vi "HFRR ADV v038 new software.vi"() -> ()   [LabVIEW 2025] (continued)
            n2186 = String Subset(string=w2638, length (rest)=9 ("length (rest)")) -> (substring=w2640:string)  [unwired: 1 in]
            n2187 = String Subset(string=w2615, length (rest)=6 ("length (rest)")) -> (substring=w2617:string)  [unwired: 1 in]
            n2188 = String Subset(string=w2633, length (rest)=9 ("length (rest)")) -> (substring=w2635:string)  [unwired: 1 in]
            n2189 = String Subset(string=w2611, length (rest)=6 ("length (rest)")) -> (substring=w2613:string)  [unwired: 1 in]
            n2190 = String Subset(string=w2628, length (rest)=9 ("length (rest)")) -> (substring=w2630:string)  [unwired: 1 in]
            n2191 = String Subset(string=w2607, length (rest)=6 ("length (rest)")) -> (substring=w2609:string)  [unwired: 1 in]
            n2192 = String Subset(string=w2623, length (rest)=9 ("length (rest)")) -> (substring=w2625:string)  [unwired: 1 in]
            n2193 = Fract/Exp String To Number(string=w2621) -> (number=w2601:dbl)  [unwired: 3 in, 1 out]
            n2194 = Fract/Exp String To Number(string=w2640) -> (number=w2641:dbl)  [unwired: 3 in, 1 out]
            n2195 = Fract/Exp String To Number(string=w2617) -> (number=w2600:dbl)  [unwired: 3 in, 1 out]
            n2196 = Fract/Exp String To Number(string=w2635) -> (number=w2636:dbl)  [unwired: 3 in, 1 out]
            n2197 = Fract/Exp String To Number(string=w2613) -> (number=w2599:dbl)  [unwired: 3 in, 1 out]
            n2198 = Fract/Exp String To Number(string=w2630) -> (number=w2631:dbl)  [unwired: 3 in, 1 out]
            n2199 = Fract/Exp String To Number(string=w2609) -> (number=w2598:dbl)  [unwired: 3 in, 1 out]
            n2200 = Fract/Exp String To Number(string=w2625) -> (number=w2626:dbl)  [unwired: 3 in, 1 out]
            n2201 = local write "sample1"(w2601) -> ()
            n2202 = local write "freq1"(w2641) -> ()
            n2203 = local write "sample2"(w2600) -> ()
            n2204 = local write "freq2"(w2636) -> ()
            n2205 = local write "sample3"(w2599) -> ()
            n2206 = local write "freq3"(w2631) -> ()
            n2207 = local write "sample4"(w2598) -> ()
            n2208 = local write "freq 4"(w2626) -> ()
          }
        }
      }
    }
    n2209 = case shown="True" w2199 {
      selector: w2199 -> [_ w2218]
      frame False {
      }
      frame True {
        n2210 = Not(x=w2218) -> (.not. x?=w2214:bool)
        n2211 = local write "service 3"(w2214) -> ()
        n2212 = local write "OPEN 6"(w2214) -> ()
        n2213 = call <vilib>:"System Exec.vi"("wait until completion? (T)"=TRUE, "command line"="C:\\LAB-IQ\\Scar View.exe") -> ("error out"=→"error out 5":errorcluster)  [unwired: 6 in, 3 out]
      }
    }
    n2214 = case shown="\"Acquire\", Default" w2208 {
      frame "Acquire", Default {
        # "Elapsed time\ncof\nstroke\nAir temp\nTemp\nHumidity"
        n2215 = disable-structure shown="Disabled" {
          frame Disabled {
            n2216 = local read "Flag"() -> (w2917:dbl)
            n2217 = local read "RUN"() -> (w2914:bool)
            n2218 = Not(x=w2914) -> (.not. x?=w2913:bool)
            n2219 = Equal?(x=w2917, y=10.0) -> (x = y?=w2915:bool)
            n2220 = And(x=w2915, y=w2913) -> (x .and. y?=w2912:bool)
            n2221 = case shown="True" w2912 {
              frame False {
              }
              frame True {
                w2918 = FALSE ("Heater Button")
                n2222 = local write "Humidity"(w2918) -> ()
                n2223 = local write "Heater Button"(w2918) -> ()
              }
            }
          }
          frame Enabled {
          }
        }
        n2224 = disable-structure shown="Disabled" {
          frame Disabled {
            n2225 = case shown="True" {
              selector: _ -> [_ _]
              frame False {
              }
              frame True {
                w2967 = TRUE ("Heater")
                n2226 = local write "Humidity"(w2967) -> ()
                n2227 = local write "Heater Button"(w2967) -> ()
                n2228 = local read "TEST STANDARD"() -> (w2970:T3)
                n2229 = local read "TEST STANDARD"() -> (w2965:T3)
                n2230 = Equal?(x=w2970, y=enum16{"ASTM D6079", "ISO 12156", "Custom"}."ISO 12156" ("Test Standard")) -> (x = y?=w2968:bool)
                n2231 = Equal?(x=w2965, y=enum16{"ASTM D6079", "ISO 12156", "Custom"}."ASTM D6079" ("Test Standard")) -> (x = y?=w2964:bool)
                n2232 = case shown="True" w2968 {
                  frame False {
                  }
                  frame True {
                    n2233 = local write "airtempflg"(FALSE ("airtempflg")) -> ()
                    n2234 = local write item#-1(TRUE ("Heater")) -> ()
                  }
                }
                n2235 = case shown="True" w2964 {
                  frame False {
                  }
                  frame True {
                    n2236 = local write "airtempflg"(TRUE ("airtempflg")) -> ()
                    n2237 = local write item#-1(FALSE ("Heater")) -> ()
                  }
                }
              }
            }
          }
          frame Enabled {
          }
        }
        n2238 = stacked-sequence {
          frame #0 {
            n2239 = case shown="True" "RST FF" {
              frame False {
              }
              frame True {
                w2984 = 0.0 ("X Scale.Range:Maximum")
                n2240 = property on="Frictional Force ( N )" class="WFChart (strict)"("XScale.Maximum"=600.0 ("X Scale.Range:Maximum"), "XScale.Minimum"=w2984, "YScale.Maximum"=10.0 ("Y Scale.Range:Maximum"), "YScale.Minimum"=w2984) -> ()  [unwired: 2 in, 2 out]
              }
            }
          }
          frame #1 {
            n2241 = case shown="True" "RST TEMP" {
              frame False {
              }
              frame True {
                n2242 = property on="Temperature ( Deg C )" class="WFChart (strict)"("XScale.Minimum"=0.0 ("X Scale.Range:Minimum"), "XScale.Maximum"=600.0 ("X Scale.Range:Maximum"), "YScale.Minimum"=0.0 ("Y Scale.Range:Minimum"), "YScale.Maximum"=100.0 ("Y Scale.Range:Maximum")) -> ()  [unwired: 2 in, 2 out]
              }
            }
          }
          frame #2 {
            n2243 = case shown="True" "RSTCOF" {
              frame False {
              }
              frame True {
                n2244 = property on="Coefficient of Friction" class="WFChart (strict)"("XScale.Minimum"=0.0 ("X Scale.Range:Minimum"), "XScale.Maximum"=600.0 ("X Scale.Range:Maximum"), "YScale.Maximum"=1.0 ("X Scale.Range:Minimum"), "YScale.Minimum"=0.0 ("X Scale.Range:Minimum")) -> ()  [unwired: 2 in, 2 out]
              }
            }
          }
          frame #3 {
            n2245 = case shown="True" "RSTCOF 2" {
              frame False {
              }
              frame True {
                (unwired) 100.0 ("Y Scale.Range:Maximum")
                (unwired) 0.0 ("Y Scale.Range:Minimum")
                (unwired) 600.0 ("X Scale.Range:Maximum")
                (unwired) 0.0 ("X Scale.Range:Minimum")
              }
            }
          }
          frame #4 {
            n2246 = case shown="True" "RSTCOF 3" {
              frame False {
              }
              frame True {
                n2247 = property on="Electrical Contact Resistance ( % )" class="WFChart (strict)"("XScale.Minimum"=0.0 ("X Scale.Range:Minimum"), "XScale.Maximum"=600.0 ("X Scale.Range:Maximum"), "YScale.Minimum"=0.0 ("Y Scale.Range:Minimum"), "YScale.Maximum"=100.0 ("Y Scale.Range:Maximum")) -> ()  [unwired: 2 in, 2 out]
              }
            }
          }
        }
        n2248 = local read "RUN"() -> (w2907:bool)
        n2249 = case shown="False" w2907 {
          frame False {
          }
          frame True {
          }
        }
        n2250 = local read "RUN"() -> (w2911:bool)
        n2251 = case shown="False" w2911 {
          tunnel: [FALSE ("TEST RUNNING") TRUE ("TEST RUNNING")] -> w2910
          frame False {
            w3003 = 0.0 ("Flag")
            n2252 = local write "Elapsed time"(0.0 ("elapsedtime")) -> ()
            n2253 = local write "Time Remaining"(w3003) -> ()
            n2254 = local write "Flag"(w3003) -> ()
            n2255 = local write "Remaining Time"(w3003) -> ()
          }
          frame True {
            n2256 = local write "Flag"(10.0 ("Flag")) -> ()
          }
        }
        n2257 = local read "AIR TEMP"() -> (w2905:dbl)
        n2258 = Greater Or Equal?(x=w2905, y=15.0) -> (x >= y?=w2906:bool)
        "powstat" <- w2906
        n2259 = case shown="True" "Save & Continue" {
          frame False {
          }
          frame True {
            n2260 = local read "USER ID"() -> (w3311:string)
            n2261 = local read "FILE"() -> (w3319:string)
            n2262 = String Length(string=w3319) -> (length=w3317:i32)
            n2263 = String Length(string=w3311) -> (length=w3314:i32)
            n2264 = Greater?(x=w3317, y=0) -> (0:w3316:bool)
            n2265 = Greater?(x=w3314, y=0) -> (0:w3313:bool)
            n2266 = And(x=w3316, y=w3313) -> (x .and. y?=w3312:bool)
            n2267 = case shown="True" w3312 {
              frame False {
                n2268 = stacked-sequence {
                  frame #0 {
                    n2269 = One Button Dialog(message="Please Enter a File Name and Operator ID to save data !", button name ("OK")="Ok") -> ()  [unwired: 1 out]
                  }
                  frame #1 {
                    n2270 = local write "Save & Continue"(FALSE ("OK Button")) -> ()
                  }
                }
                n2271 = local write "Save & Continue"(FALSE ("OK Button")) -> ()
              }
              frame True {
                n2272 = stacked-sequence {
                  frame #0 {
                    n2273 = local read "FILE"() -> (w3325:string)
                    n2274 = call "file check.vi"("file name in"=w3325) -> ("file name out"=w3324:string)  [unwired: 9 in, 1 out]
                    n2275 = call <vilib>:"Application Directory.vi"() -> ("Application Directory"=w3335:path)
                    n2276 = Build Path(base path=w3335, name or relative path="data") -> (appended path=w3334:path)
                    n2277 = call <vilib>:"Trim Whitespace.vi"("string"=w3324) -> ("trimmed string"=w3332:string)  [unwired: 1 in]
                    n2278 = call <vilib>:"Trim Whitespace.vi"("string"=w3324) -> ("trimmed string"=w3333:string)  [unwired: 1 in]
                    n2279 = List Folder(path=w3334) -> (folder names=w3330:string[])  [unwired: 3 in, 3 out]
                    n2280 = Match Pattern(string=w3332, regular expression="_(") -> (before substring=w3329:string)  [unwired: 1 in, 3 out]
                    n2281 = for {
                      tunnel: w3330 -> [w3344] mode=indexing
                      tunnel: w3329 -> [w3342]
                      shift-right: [w3340] -> w3327
                      shift-left: bool[] [] -> [w3341]
                      n2282 = Match Pattern(string=w3344, regular expression="_(") -> (before substring=w3343:string)  [unwired: 1 in, 3 out]
                      n2283 = Equal?(x=w3343, y=w3342) -> (x = y?=w3339:bool)
                      n2284 = case shown="True" w3339 {
                        tunnel: w3339 -> [_ w3347]
                        tunnel: w3341 -> [w3346 w3349]
                        tunnel: [w3346 w3348] -> w3340
                        frame False {
                        }
                        frame True {
                          n2285 = Insert Into Array(array=w3349, new element=w3347) -> (w3348:bool[])  [unwired: 1 in]
                        }
                      }
                    }
                    n2286 = Equal?(x=w3330, y=w3329) -> (x = y?=w3338:bool[])
                    n2287 = Or Array Elements(Boolean array=w3338) -> (logical OR=w3337:bool)
                    n2288 = Array Size(array=w3327) -> (size(s)=w3326:i32)
                    n2289 = case shown="True" w3337 {
                      tunnel: w3333 -> [_ w3357]
                      tunnel: w3326 -> [_ w3350]
                      frame False {
                      }
                      frame True {
                        n2290 = Number To Decimal String(number=w3350) -> (decimal integer string=w3353:string)  [unwired: 1 in]
                        n2291 = Search/Split String(string=w3357, search string/char (-)="_(" ("regular expression")) -> (substring before match=w3355:string)  [unwired: 1 in, 2 out]
                        n2292 = Concatenate Strings(w3355, "_(" ("regular expression"), w3353, ")" ("regular expression")) -> (w3351:string)
                        n2293 = local write "FILE"(w3351) -> ()
                      }
                    }
                  }
                  frame #1 {
                    w3360 = 0.0
                    w3373 = cluster{"y":dbl, dbl, "y":dbl}[] [] ("History Data")
                    w3374 = FALSE ("Heater Button")
                    (unwired) ")!" ("string")
                    (unwired) ")" ("string")
                    w3372 = dbl[] [] ("History Data")
                    w3378 = "\r"
                    # "C:\\WinDucom\\Data\\"
                    # "C:\\LAB-IQ-NXT\\data"
                    n2294 = local write "Humidity ( %RH )"(w3360) -> ()
                    n2295 = local write "Frequency ( Hz )"(w3360) -> ()
                    n2296 = local write "Stroke 3"(w3360) -> ()
                    n2297 = local write "speedop"(0.0 ("PIDclk 2")) -> ()
                    n2298 = local write "Set Temp 2"(65.0 ("Set Temp 2")) -> ()
                    n2299 = local write "AIR TEMP"(w3360) -> ()
                    n2300 = local write "clk"(0.0 ("clk")) -> ()
                    n2301 = local write "Stroke 4"(w3360) -> ()
                    n2302 = local write "COF 2"(w3360) -> ()
                    n2303 = local write "TEMP"(w3360) -> ()
                    n2304 = local write "ecr 3"(w3360) -> ()
                    n2305 = local write "FF 3"(w3360) -> ()
                    n2306 = local write "FF 2"(w3360) -> ()
                    n2307 = property on="Humidity ( %RH ) 2" class="WFChart (strict)"("History Data"=w3372) -> ()  [unwired: 2 in, 2 out]
                    n2308 = property on="Coefficient of Friction" class="WFChart (strict)"("History Data"=w3372) -> ()  [unwired: 2 in, 2 out]
                    n2309 = property on="Coefficient of Friction" class="WFChart (strict)"("History Data"=w3372) -> ()  [unwired: 2 in, 2 out]
                    n2310 = property on="Frictional Force ( N )" class="WFChart (strict)"("History Data"=w3372) -> ()  [unwired: 2 in, 2 out]
                    n2311 = property on="Electrical Contact Resistance ( % )" class="WFChart (strict)"("History Data"=w3372) -> ()  [unwired: 2 in, 2 out]
                    n2312 = property on="Electrical Contact Resistance ( % )" class="WFChart (strict)"("History Data"=w3372) -> ()  [unwired: 2 in, 2 out]
                    n2313 = property on="Temperature ( Deg C )" class="WFChart (strict)"("History Data"=w3372) -> ()  [unwired: 2 in, 2 out]
                    n2314 = property on="Frictional Force ( N )" class="WFChart (strict)"("History Data"=w3372) -> ()  [unwired: 2 in, 2 out]
                    n2315 = property on="Coefficient of Friction" class="WFChart (strict)"("History Data"=w3372) -> ()  [unwired: 2 in, 2 out]
                    n2316 = property on="Frictional Force ( N )" class="WFChart (strict)"("History Data"=w3372) -> ()  [unwired: 2 in, 2 out]
                    n2317 = property on="Electrical Contact Resistance ( % )" class="WFChart (strict)"("History Data"=w3372) -> ()  [unwired: 2 in, 2 out]
                    n2318 = property on="Temperature ( Deg C )" class="WFChart (strict)"("History Data"=w3372) -> ()  [unwired: 2 in, 2 out]
                    n2319 = property on="Stroke ( mm )" class="WFChart (strict)"("History Data"=w3373) -> ()  [unwired: 2 in, 2 out]
                    n2320 = property on="Stroke ( mm )" class="WFChart (strict)"("History Data"=w3373) -> ()  [unwired: 2 in, 2 out]
                    n2321 = local write "Humidity"(w3374) -> ()
                    n2322 = local write "Heater Button"(w3374) -> ()
                    n2323 = local read "FILE"() -> (w3368:string)
                    n2324 = disable-structure shown="Enabled" {
                      disable-tunnel: [w3412 _] -> w3359
                      frame Enabled {
                        n2325 = local read "NORMAL LOAD"() -> (w3412:dbl)
                      }
                      frame Disabled {
                      }
                    }
                    n2326 = call "file check.vi"("file name in"=w3368) -> ("error out"=w3371:errorcluster, "file name out"=w3365:string)  [unwired: 9 in]
                    n2327 = call "FILE PATH CREATION.vi"("error in"=w3371, "FILE NAME :"=w3365) -> ("FILE OUT"=w3364:path)  [unwired: 8 in, 1 out]
                    n2328 = Concatenate Strings(w3365, ".dgf" ("Substring")) -> (w3370:string)
                    n2329 = Concatenate Strings(w3365, ".duf" ("Substring")) -> (w3366:string)
                    n2330 = Multiply(x=w3359, y=1.0) -> (x*y=w3391:dbl)
                    n2331 = Build Path(base path=w3364, name or relative path=w3370) -> (appended path=w3363:path)
                    n2332 = Build Path(base path=w3364, name or relative path=w3366) -> (appended path=w3362:path)
                    n2333 = Number To Fractional String(number=w3391, width (-)=i16 5, precision (6)=i16 2) -> (F-format string=w3399:string)  [unwired: 1 in]
                    n2334 = local read "tested by"() -> (w3358:string)
                    n2335 = local read "Fuel Discription :"() -> (w3387:string)
                    n2336 = local read "Batch Ref Num :"() -> (w3376:string)
                    n2337 = Get Date/Time String(date format (0)=enum16{"short", "long", "abbreviated"}."short") -> (date string=w3410:string, time string=w3407:string)  [unwired: 2 in]
                    n2338 = local read "Remarks :"() -> (w3386:string)
                    n2339 = Concatenate Strings("Load :- " ("Substring"), w3399, " grams ," ("Substring")) -> (w3398:string)
                    n2340 = local read "String 41"() -> (w3379:string)
                    n2341 = Concatenate Strings(w3387) -> (w3388:string)
                    n2342 = Concatenate Strings(w3376) -> (w3375:string)
                    n2343 = Concatenate Strings(w3358) -> (w3382:string)
                    n2344 = Concatenate Strings("(" ("Substring"), w3410, ")" ("Substring"), w3407) -> (w3381:string)
                    "concatenated string" <- w3381
                    n2345 = Concatenate Strings(w3386, "," ("string")) -> (w3385:string)
                    n2346 = Concatenate Strings("  TIME;      COF;       STROKE;     AIR TEMP;  TEMP;  HUMIDITY;  ECR; PID-OUT; FREQUENCY" ("Substring"), "\r") -> (w3394:string)
                    n2347 = Concatenate Strings(w3379, w3378, "Fuel Discription :-" ("Substring"), w3388, w3378, w3398, w3378, "Batch Ref Num :-" ("Substring"), w3375, w3378, " Remarks :- " ("Substring"), w3385, w3378, " Date :- " ("Substring"), w3381, w3378, "Tested By :-" ("Substring"), w3382) -> (w3392:string)
                    "REMARKS" <- w3392
                    n2348 = call <vilib>:"Write Characters To File.vi"("append to file? (new file:F)"=FALSE, "character string"=w3394, "file path (dialog if empty)"=w3363) -> ()  [unwired: 2 in, 1 out]
                    n2349 = call <vilib>:"Write Characters To File.vi"("append to file? (new file:F)"=FALSE, "character string"=w3392, "file path (dialog if empty)"=w3362) -> ()  [unwired: 2 in, 1 out]
                  }
                  frame #2 {
                    n2350 = local write "Cycles elapsed"(0 ("Cycles elapsed")) -> ()
                    n2351 = local write "cyclecount"(0 ("cyclecount")) -> ()
                    n2352 = local write "Save & Continue"(FALSE ("OK")) -> ()
                    n2353 = local write "autostrtflg"(TRUE ("autostrtflg")) -> ()
                    n2354 = local write "Save"(FALSE ("Save")) -> ()
                    n2355 = Get Date/Time In Seconds() -> (seconds since 1Jan1904=w3417:timestamp)
                    n2356 = To Double Precision Float(number=w3417) -> (double precision float=w3416:dbl)
                    n2357 = local write "acq timer"(w3416) -> ()
                    n2358 = One Button Dialog(message="Please ensure sample is mounted properly and machine is ready in all aspects for testing !", button name ("OK")="Ok") -> ()  [unwired: 1 out]
                  }
                  frame #3 {
                    n2359 = stacked-sequence {
                      frame #0 {
                        n2360 = local write "Main Dashboard Buttons"(T1."Dashboard" ("Main Dashboard Buttons")) -> ()
                        n2361 = local write "Main Tab"(T2."Acquire" ("Main Tab")) -> ()
                      }
                      frame #1 {
                        n2362 = local write "EVENT LOG"("" ("EVENT LOG")) -> ()
                      }
                      frame #2 {
                        n2363 = Wait (ms)(milliseconds to wait=u32 50) -> ()  [unwired: 1 out]
                      }
                      frame #3 {
                        n2364 = disable-structure shown="Disabled" {
                          frame Disabled {
                            n2365 = local read "EVENT LOG"() -> (w3429:string)
                            n2366 = call "Event Log.vi"("Content"="Test Details", "EVENT LOG"=w3429) -> ("EVENT LOG"=w3428:string)  [unwired: 8 in, 1 out]
                            n2367 = local write "EVENT LOG"(w3428) -> ()
                          }
                          frame Enabled {
                          }
                        }
                      }
                      frame #4 {
                        n2368 = Wait (ms)(milliseconds to wait=u32 50) -> ()  [unwired: 1 out]
                      }
                      frame #5 {
                        n2369 = local read "FILE"() -> (w3431:string)
                        n2370 = Concatenate Strings("File Name :" ("Content"), w3431) -> (w3432:string)
                        n2371 = local read "EVENT LOG"() -> (w3435:string)
                        n2372 = call "Event Log.vi"("Content"=w3432, "EVENT LOG"=w3435) -> ("EVENT LOG"=w3434:string)  [unwired: 8 in, 1 out]
                        n2373 = local write "EVENT LOG"(w3434) -> ()
                      }
                      frame #6 {
                        n2374 = Wait (ms)(milliseconds to wait=u32 50) -> ()  [unwired: 1 out]
                      }
                      frame #7 {
                        n2375 = local read "Batch Ref Num :"() -> (w3437:string)
                        n2376 = Concatenate Strings("Batch Ref No :" ("Content"), w3437) -> (w3438:string)
                        n2377 = local read "EVENT LOG"() -> (w3441:string)
                        n2378 = call "Event Log.vi"("Content"=w3438, "EVENT LOG"=w3441) -> ("EVENT LOG"=w3440:string)  [unwired: 8 in, 1 out]
                        n2379 = local write "EVENT LOG"(w3440) -> ()
                      }
                      frame #8 {
                        n2380 = Wait (ms)(milliseconds to wait=u32 50) -> ()  [unwired: 1 out]
                      }
                      frame #9 {
                        n2381 = local read "tested by"() -> (w3443:string)
                        n2382 = Concatenate Strings("Tested By :" ("Content"), w3443) -> (w3444:string)
                        n2383 = local read "EVENT LOG"() -> (w3447:string)
                        n2384 = call "Event Log.vi"("Content"=w3444, "EVENT LOG"=w3447) -> ("EVENT LOG"=w3446:string)  [unwired: 8 in, 1 out]
                        n2385 = local write "EVENT LOG"(w3446) -> ()
                      }
                      frame #10 {
                        n2386 = Wait (ms)(milliseconds to wait=u32 50) -> ()  [unwired: 1 out]
                      }
                      frame #11 {
                        n2387 = local read "TEST STANDARD"() -> (w3450:T3)
                        n2388 = case shown="\"ASTM D6079\", Default" w3450 {
                          tunnel: ["ASTM D6079" "ISO 12156" "CEC F-096-A-06" "Custom"] -> w3449
                          frame "ASTM D6079", Default {
                          }
                          frame "ISO 12156" {
                          }
                          frame "CEC F-096-A-06" {
                          }
                          frame "Custom" {
                          }
                        }
                        n2389 = Concatenate Strings("Test Standard :" ("Content"), w3449) -> (w3451:string)
                        n2390 = local read "EVENT LOG"() -> (w3454:string)
                        n2391 = call "Event Log.vi"("Content"=w3451, "EVENT LOG"=w3454) -> ("EVENT LOG"=w3453:string)  [unwired: 8 in, 1 out]
                        n2392 = local write "EVENT LOG"(w3453) -> ()
                      }
                      frame #12 {
                        n2393 = Wait (ms)(milliseconds to wait=u32 50) -> ()  [unwired: 1 out]
                      }
                      frame #13 {
                        n2394 = local read "Fuel Discription :"() -> (w3460:string)
                        n2395 = Concatenate Strings("Fuel Description :" ("Content"), w3460) -> (w3461:string)
                        n2396 = local read "EVENT LOG"() -> (w3464:string)
                        n2397 = call "Event Log.vi"("Content"=w3461, "EVENT LOG"=w3464) -> ("EVENT LOG"=w3463:string)  [unwired: 8 in, 1 out]
                        n2398 = local write "EVENT LOG"(w3463) -> ()
                      }
                      frame #14 {
                        n2399 = Wait (ms)(milliseconds to wait=u32 50) -> ()  [unwired: 1 out]
                      }
                      frame #15 {
                        n2400 = local read "Remarks :"() -> (w3466:string)
                        n2401 = Concatenate Strings("Remarks :" ("Content"), w3466) -> (w3467:string)
                        n2402 = local read "EVENT LOG"() -> (w3470:string)
                        n2403 = call "Event Log.vi"("Content"=w3467, "EVENT LOG"=w3470) -> ("EVENT LOG"=w3469:string)  [unwired: 8 in, 1 out]
                        n2404 = local write "EVENT LOG"(w3469) -> ()
                      }
                      frame #16 {
                        n2405 = Wait (ms)(milliseconds to wait=u32 50) -> ()  [unwired: 1 out]
                      }
                      frame #17 {
                        n2406 = local read "USER ID"() -> (w3472:string)
                        n2407 = Concatenate Strings("Operator ID :" ("Content"), w3472) -> (w3474:string)
                        n2408 = local read "EVENT LOG"() -> (w3476:string)
                        n2409 = call "Event Log.vi"("Content"=w3474, "EVENT LOG"=w3476) -> ("EVENT LOG"=w3475:string)  [unwired: 8 in, 1 out]
                        n2410 = local write "EVENT LOG"(w3475) -> ()
                      }
                      frame #18 {
                        n2411 = Wait (ms)(milliseconds to wait=u32 50) -> ()  [unwired: 1 out]
                      }
                      frame #19 {
                        n2412 = disable-structure shown="Disabled" {
                          frame Disabled {
                            n2413 = local read "EVENT LOG"() -> (w3480:string)
                            n2414 = call "Event Log.vi"("Content"="Test Parameter", "EVENT LOG"=w3480) -> ("EVENT LOG"=w3479:string)  [unwired: 8 in, 1 out]
                            n2415 = local write "EVENT LOG"(w3479) -> ()
                          }
                          frame Enabled {
                          }
                        }
                      }
                      frame #20 {
                        n2416 = Wait (ms)(milliseconds to wait=u32 50) -> ()  [unwired: 1 out]
                      }
                      frame #21 {
                        n2417 = local read "Set Hz"() -> (w3484:dbl)
                        n2418 = Number To Fractional String(number=w3484, precision (6)=i16 2) -> (F-format string=w3483:string)  [unwired: 2 in]
                        n2419 = Concatenate Strings("Set Frequency [Hz] :" ("Content"), w3483) -> (w3486:string)
                        n2420 = local read "EVENT LOG"() -> (w3488:string)
                        n2421 = call "Event Log.vi"("Content"=w3486, "EVENT LOG"=w3488) -> ("EVENT LOG"=w3487:string)  [unwired: 8 in, 1 out]
                        n2422 = local write "EVENT LOG"(w3487) -> ()
                      }
                      frame #22 {
                        n2423 = Wait (ms)(milliseconds to wait=u32 50) -> ()  [unwired: 1 out]
                      }
                      frame #23 {
                        n2424 = local read "NORMAL LOAD"() -> (w3491:dbl)
                        n2425 = Number To Fractional String(number=w3491, precision (6)=i16 2) -> (F-format string=w3492:string)  [unwired: 2 in]
                        n2426 = Concatenate Strings("Applied Load [grams] :" ("Content"), w3492) -> (w3494:string)
                        n2427 = local read "EVENT LOG"() -> (w3496:string)
                        n2428 = call "Event Log.vi"("Content"=w3494, "EVENT LOG"=w3496) -> ("EVENT LOG"=w3495:string)  [unwired: 8 in, 1 out]
                        n2429 = local write "EVENT LOG"(w3495) -> ()
                      }
                      frame #24 {
                        n2430 = Wait (ms)(milliseconds to wait=u32 50) -> ()  [unwired: 1 out]
                      }
                      frame #25 {
                        n2431 = local read "Set Strk"() -> (w3499:dbl)
                        n2432 = Number To Fractional String(number=w3499, precision (6)=i16 2) -> (F-format string=w3500:string)  [unwired: 2 in]
                        n2433 = Concatenate Strings("Set Stroke [mm] :" ("Content"), w3500) -> (w3502:string)
                        n2434 = local read "EVENT LOG"() -> (w3504:string)
                        n2435 = call "Event Log.vi"("Content"=w3502, "EVENT LOG"=w3504) -> ("EVENT LOG"=w3503:string)  [unwired: 8 in, 1 out]
                        n2436 = local write "EVENT LOG"(w3503) -> ()
                      }
                      frame #26 {
                        n2437 = Wait (ms)(milliseconds to wait=u32 50) -> ()  [unwired: 1 out]
                      }
                      frame #27 {
                        n2438 = local read "Set Temp"() -> (w3507:dbl)
                        n2439 = Number To Fractional String(number=w3507, precision (6)=i16 2) -> (F-format string=w3508:string)  [unwired: 2 in]
                        n2440 = Concatenate Strings("Set Temperature [deg C] :" ("Content"), w3508) -> (w3510:string)
                        n2441 = local read "EVENT LOG"() -> (w3512:string)
                        n2442 = call "Event Log.vi"("Content"=w3510, "EVENT LOG"=w3512) -> ("EVENT LOG"=w3511:string)  [unwired: 8 in, 1 out]
                        n2443 = local write "EVENT LOG"(w3511) -> ()
                      }
                      frame #28 {
                        n2444 = Wait (ms)(milliseconds to wait=u32 50) -> ()  [unwired: 1 out]
                      }
                      frame #29 {
                        n2445 = local read "Set Rh"() -> (w3515:dbl)
                        n2446 = Number To Fractional String(number=w3515, precision (6)=i16 2) -> (F-format string=w3516:string)  [unwired: 2 in]
                        n2447 = Concatenate Strings("Set Humidity [%RH] :" ("Content"), w3516) -> (w3518:string)
                        n2448 = local read "EVENT LOG"() -> (w3520:string)
                        n2449 = call "Event Log.vi"("Content"=w3518, "EVENT LOG"=w3520) -> ("EVENT LOG"=w3519:string)  [unwired: 8 in, 1 out]
                        n2450 = local write "EVENT LOG"(w3519) -> ()
                      }
                      frame #30 {
                        n2451 = Wait (ms)(milliseconds to wait=u32 50) -> ()  [unwired: 1 out]
                      }
                      frame #31 {
                        n2452 = local read "test time"() -> (w3523:dbl)
                        n2453 = Number To Fractional String(number=w3523, precision (6)=i16 1) -> (F-format string=w3524:string)  [unwired: 2 in]
                        n2454 = Concatenate Strings("Test Duration [mins] :" ("Content"), w3524) -> (w3526:string)
                        n2455 = local read "EVENT LOG"() -> (w3528:string)
                        n2456 = call "Event Log.vi"("Content"=w3526, "EVENT LOG"=w3528) -> ("EVENT LOG"=w3527:string)  [unwired: 8 in, 1 out]
                        n2457 = local write "EVENT LOG"(w3527) -> ()
                      }
                      frame #32 {
                        w3529 = dbl[] [] ("History Data")
                        w3530 = cluster{"y":dbl, dbl, "y":dbl}[] [] ("History Data")
                        w3531 = FALSE ("Visible")
                        n2458 = property on="Stroke ( mm )" class="WFChart (strict)"("History Data"=w3530) -> ()  [unwired: 2 in, 2 out]
                        n2459 = property on="Humidity ( %RH ) 2" class="WFChart (strict)"("History Data"=w3529) -> ()  [unwired: 2 in, 2 out]
                        n2460 = property on="Temperature ( Deg C )" class="WFChart (strict)"("History Data"=w3529) -> ()  [unwired: 2 in, 2 out]
                        n2461 = property on="Electrical Contact Resistance ( % )" class="WFChart (strict)"("History Data"=w3529) -> ()  [unwired: 2 in, 2 out]
                        n2462 = property on="Coefficient of Friction" class="WFChart (strict)"("History Data"=w3529) -> ()  [unwired: 2 in, 2 out]
                        n2463 = property on="Frictional Force ( N )" class="WFChart (strict)"("History Data"=w3529) -> ()  [unwired: 2 in, 2 out]
                        n2464 = property on="Coefficient of Friction" class="WFChart (strict)"("History Data"=w3529) -> ()  [unwired: 2 in, 2 out]
                        n2465 = property on="Frictional Force ( N )" class="WFChart (strict)"("History Data"=w3529) -> ()  [unwired: 2 in, 2 out]
                        n2466 = property on="Electrical Contact Resistance ( % )" class="WFChart (strict)"("History Data"=w3529) -> ()  [unwired: 2 in, 2 out]
                        n2467 = property on="Stroke ( mm )" class="WFChart (strict)"("History Data"=w3530) -> ()  [unwired: 2 in, 2 out]
                        n2468 = property on="Temperature ( Deg C )" class="WFChart (strict)"("History Data"=w3529) -> ()  [unwired: 2 in, 2 out]
                        n2469 = property on="Service Password Log" class="Str"("Visible"=w3531) -> ()  [unwired: 2 in, 2 out]
                        n2470 = property on="Password 3" class="Clust (strict)"("Visible"=w3531) -> ()  [unwired: 2 in, 2 out]
                      }
                    }
                    "TEST FILE NAM,E SAVED" <- TRUE ("TEST FILE NAM,E SAVED")
                  }
                }
              }
            }
          }
        }
        n2471 = local write "Test \nStatus"(w2910) -> ()
        n2472 = local write "Save"(w2910) -> ()
        n2473 = local read "Main Tab"() -> (w2904:T2)
        n2474 = case shown="True" w2907 {
          frame False {
            n2475 = local read "Rt 3"() -> (w2975:bool)
            n2476 = case shown="True" w2975 {
              frame False {
              }
              frame True {
                n2477 = local write "Rt 3"(FALSE ("Rt 3")) -> ()
              }
            }
            "Rt" <- TRUE ("Rt")
            "Rt 2" <- FALSE ("Rt")
          }
          frame True {
            n2478 = local read "Rt"() -> (w2981:bool)
            n2479 = local write "Rt 2"(TRUE ("Rt 2")) -> ()
            n2480 = case shown="True" w2981 {
              frame False {
              }
              frame True {
                n2481 = local write "Rt"(FALSE ("Rt")) -> ()
              }
            }
            "Rt 3" <- TRUE ("Rt 3")
          }
        }
        n2482 = case shown="\"Acquire\"" w2904 {
          tunnel: w2906 -> [_ w3010]
          frame Default {
            w3009 = 0.0 ("output")
            n2483 = local write "PID-out"(w3009) -> ()
            n2484 = local write "Frequency ( Hz )"(w3009) -> ()
            n2485 = local write "STROKE Initialize"(TRUE ("STROKE Initialize")) -> ()
          }
          frame "Acquire" {
            n2486 = stacked-sequence {
              frame #0 {
                n2487 = local read "Auto Start Test"() -> (w3012:bool)
                n2488 = case shown="True" w3012 {
                  tunnel: "RUN" -> [w3033 w3036]
                  tunnel: [w3033 w3035] -> w3013
                  frame False {
                  }
                  frame True {
                    n2489 = local read "Auto Start Temp"() -> (w3034:bool)
                    n2490 = Or(x=w3036, y=w3034) -> (x .or. y?=w3035:bool)
                  }
                }
                n2491 = local read "clk"() -> (w3032:dbl)
                n2492 = local read "Save"() -> (w3028:bool)
                n2493 = Equal?(x=w3032, y=0.0) -> (x = y?=w3029:bool)
                n2494 = And(x=w3029, y=w3028) -> (x .and. y?=w3030:bool)
                n2495 = Not(x="Engage") -> (.not. x?=w3019:bool)
                n2496 = case shown="False" w3013 {
                  tunnel: [0.0 w3059] -> w3015
                  frame False {
                    (unwired) TRUE ("Visible")
                    n2497 = local read "Auto Start Test"() -> (w3040:bool)
                    n2498 = local write "Start Time"(TRUE ("Start Time")) -> ()
                    n2499 = property on="Stroke 2" class="DigNum (strict)"("Visible"=FALSE) -> ()  [unwired: 2 in, 2 out]
                    n2500 = case shown="False" w3040 {
                      frame False {
                        n2501 = property on="Heater Button" class="Bool (strict)"("DisabledEnum"=T19."Enabled" ("Disabled")) -> ()  [unwired: 2 in, 2 out]
                        n2502 = property on="Humidity" class="Bool (strict)"("DisabledEnum"=T19."Enabled" ("Disabled")) -> ()  [unwired: 2 in, 2 out]
                      }
                      frame True {
                      }
                    }
                    n2503 = case shown="False" "TestCompFlg" {
                      frame False {
                        n2504 = local read "StartFlg"() -> (w3048:bool)
                        n2505 = case shown="True" w3048 {
                          frame False {
                          }
                          frame True {
                            n2506 = stacked-sequence {
                              frame #0 {
                                n2507 = local read "EVENT LOG"() -> (w3052:string)
                                n2508 = call "Event Log.vi"("Content"="Test was interrupted", "EVENT LOG"=w3052) -> ("EVENT LOG"=w3053:string)  [unwired: 8 in, 1 out]
                                n2509 = local write "EVENT LOG"(w3053) -> ()
                                n2510 = property on="RUN" class="Bool (strict)"("Visible"=TRUE) -> ()  [unwired: 2 in, 2 out]
                                n2511 = property on="Auto Start Test" class="Bool (strict)"("Visible"=TRUE) -> ()  [unwired: 2 in, 2 out]
                              }
                              frame #1 {
                                w3055 = FALSE ("StartFlg")
                                n2512 = property on="Heater Button" class="Bool (strict)"("Val(Sgnl)"=FALSE ("Value (Signaling)")) -> ()  [unwired: 2 in, 2 out]
                                n2513 = local write "Heater Button"(w3055) -> ()
                                n2514 = local write "StartFlg"(w3055) -> ()
                                n2515 = local write "Humidity"(w3055) -> ()
                              }
                              frame #2 {
                                n2516 = local write "Due Write"("VC;0" ("Command")) -> ()
                              }
                              frame #3 {
                                n2517 = Wait (ms)(milliseconds to wait=u32 1500) -> ()  [unwired: 1 out]
                              }
                              frame #4 {
                                n2518 = local write "Due Write"("HE;0" ("Command")) -> ()
                              }
                            }
                          }
                        }
                      }
                      frame True {
                      }
                    }
                    n2519 = local write "String 14"("Test will autostart once parameters reach the set value." ("String 14")) -> ()
                  }
                  frame True {
                    (unwired) FALSE ("Visible")
                    n2520 = property on="Stroke 2" class="DigNum (strict)"("Visible"=TRUE) -> ()  [unwired: 2 in, 2 out]
                    n2521 = property on="STOP 2" class="Bool (strict)"("Disabled"=u8 2) -> ()  [unwired: 2 in, 2 out]
                    n2522 = local write "String 14"(" Running....." ("String 14")) -> ()
                    n2523 = property on="Heater Button" class="Bool (strict)"("DisabledEnum"=T19."Disabled and Grayed Out" ("Disabled")) -> ()  [unwired: 2 in, 2 out]
                    n2524 = property on="Humidity" class="Bool (strict)"("DisabledEnum"=T19."Disabled and Grayed Out" ("Disabled")) -> ()  [unwired: 2 in, 2 out]
                    n2525 = case shown="True" "Start Time" {
                      selector: "Start Time" -> [_ w3078]
                      frame False {
                      }
                      frame True {
                        n2526 = Not(x=w3078) -> (.not. x?=w3077:bool)
                        n2527 = local write "Start Time"(w3077) -> ()
                        n2528 = local read "EVENT LOG"() -> (w3079:string)
                        n2529 = call "Event Log.vi"("Content"="Test in progress", "EVENT LOG"=w3079) -> ("EVENT LOG"=w3081:string)  [unwired: 8 in, 1 out]
                        n2530 = local write "EVENT LOG"(w3081) -> ()
                      }
                    }
                    n2531 = disable-structure shown="Enabled" {
                      disable-tunnel: [w3070 w3076] -> w3059
                      frame Disabled {
                        n2532 = local read "Set Hz"() -> (w3073:dbl)
                        n2533 = call <vilib>:"Uniform White Noise Waveform.vi"() -> ("signal out"=w3072:waveform(dbl))  [unwired: 10 in, 1 out]
                        n2534 = Random Number (0-1)() -> (number: 0 to 1=w3069:dbl)
                        n2535 = Add(x=w3073, y=w3072) -> (x+y=w3071:waveform(dbl))
                        n2536 = Multiply(x=ext 0.01 ("y"), y=w3069) -> (x*y=w3067:ext)
                        n2537 = Multiply(x=w3071, y=w3067) -> (x*y=w3070:waveform(ext))
                      }
                      frame Enabled {
                        n2538 = call-poly <vilib>:"Random Number (Range).vi"("lower bound (0)"=49.89, "upper bound (100)"=50.8) -> ("number"=w3076:dbl)  [unwired: 9 in]
                      }
                    }
                    "StartFlg" <- TRUE ("StartFlg")
                  }
                }
                n2539 = case shown="True" w3030 {
                  frame False {
                  }
                  frame True {
                    n2540 = local write "clk"(10.0 ("clk")) -> ()
                    n2541 = Get Date/Time In Seconds() -> (seconds since 1Jan1904=w3084:timestamp)
                    n2542 = To Double Precision Float(number=w3084) -> (double precision float=w3082:dbl)
                    n2543 = local write "acq timer"(w3082) -> ()
                    n2544 = local write "act save time"(w3082) -> ()
                  }
                }
                n2545 = call "Elapsed Time"("Time Target (s)"="Countdown", "Reset"=w3019) -> ("Elapsed Time (s)"=w3024:dbl, "Time has Elapsed"=w3022:bool)  [unwired: 10 in, 6 out]
                "Countdown 2" <- w3024
                n2546 = Subtract(x=w3024, y=2.0) -> (x-y=w3027:dbl)
                n2547 = Less?(x=w3027, y="Countdown") -> (x < y?=w3025:bool)
                n2548 = And(x=w3025, y=w3022) -> (x .and. y?=w3021:bool)
                n2549 = case shown="True" w3021 {
                  frame False {
                  }
                  frame True {
                    (unwired) dbl[] [] ("History Data")
                    n2550 = local write "Engage"(FALSE ("Engage")) -> ()
                    n2551 = local write "RUN"(TRUE ("RUN")) -> ()
                    n2552 = local read "Humidity ( %RH )"() -> (→"Rh Before":dbl)
                  }
                }
                n2553 = local read "Test \nStatus"() -> (w3017:bool)
                n2554 = Select(t=w3015, s=w3017, f=0.0) -> (s? t:f=w3016:dbl)
                n2555 = local write "Frequency ( Hz )"(w3016) -> ()
              }
              frame #1 {
                w3107 = 1000000.0 ("x")
                # "HC;1/0\nST;VALUE"
                # "Elapsed time\ncof\nstroke\nAir temp\nTemp\nHumidity"
                # "acq timer\n\nact save time"
                # "convert to microseconds"
                n2556 = local read "COUNT"() -> (w3090:i32)
                n2557 = local read "Rate"() -> (w3103:dbl)
                n2558 = Divide(x=w3107, y=w3103) -> (x/y=w3108:dbl)
                n2559 = Greater Or Equal?(x=w3090, y=250) -> (x >= y?=w3089:bool)
                n2560 = Get Date/Time In Seconds() -> (seconds since 1Jan1904=w3110:timestamp)
                n2561 = case shown="True" w3089 {
                  frame False {
                    n2562 = local read "COUNT"() -> (w3111:i32)
                    n2563 = Increment(x=w3111) -> (x+1=w3112:i32)
                    n2564 = local write "COUNT"(w3112) -> ()
                  }
                  frame True {
                    n2565 = local write "COUNT"(0 ("COUNT")) -> ()
                  }
                }
                n2566 = local read "Samplingtime 2"() -> (w3088:dbl)
                n2567 = local read "act save time"() -> (w3105:dbl)
                n2568 = Divide(x=w3108, y=w3107) -> (x/y=w3106:dbl)
                n2569 = To Double Precision Float(number=w3110) -> (double precision float=w3099:dbl)
                n2570 = Add(x=w3105, y=w3088) -> (x+y=w3104:dbl)
                n2571 = local read "acq timer"() -> (w3109:dbl)
                n2572 = local read "COUNT"() -> (w3092:i32)
                n2573 = Greater Or Equal?(x=w3099, y=w3104) -> (x >= y?=w3087:bool)
                n2574 = Multiply(x=w3106, y=w3092) -> (x*y=w3098:dbl)
                n2575 = Subtract(x=w3099, y=w3109) -> (x-y=w3101:dbl)
                n2576 = local read "Save"() -> (w3102:bool)
                n2577 = Add(x=w3101, y=w3098) -> (x+y=w3085:dbl)
                "Elapsed time 3" <- w3085
                n2578 = And(x=w3087, y=w3102) -> (x .and. y?=w3100:bool)
                n2579 = Divide(x=w3085, y=60.0) -> (x/y=w3096:dbl)
                n2580 = local read "Test \nStatus"() -> (w3086:bool)
                n2581 = local read "clk"() -> (w3093:dbl)
                n2582 = Equal?(x=w3093, y=10.0) -> (x = y?=w3095:bool)
                n2583 = case shown="True" w3100 {
                  tunnel: w3099 -> [_ w3231]
                  tunnel: [FALSE ("Boolean 2") TRUE ("Boolean 2")] -> _
                  frame False {
                  }
                  frame True {
                    w3185 = ";" ("Substring")
                    # "Pid out/\nFreq response value"
                    n2584 = local write "act save time"(w3231) -> ()
                    n2585 = local read "FILE"() -> (w3179:string)
                    n2586 = call "file check.vi"("file name in"=w3179) -> ("error out"=w3182:errorcluster, "file name out"=w3177:string)  [unwired: 9 in]
                    n2587 = local read "LVDT STROKE"() -> (w3174:dbl)
                    n2588 = local read "Add up Stroke"() -> (w3172:dbl)
                    n2589 = call "FILE PATH CREATION.vi"("error in"=w3182, "FILE NAME :"=w3177) -> ("FILE OUT"=w3180:path)  [unwired: 8 in, 1 out]
                    n2590 = local read "STROKE Initialize"() -> (w3167:bool)
                    n2591 = Concatenate Strings(w3177, ".dgf" ("Substring")) -> (w3181:string)
                    n2592 = Subtract(x=w3174, y=w3172) -> (x-y=w3173:dbl)
                    n2593 = Absolute Value(x=w3173) -> (abs(x)=w3170:dbl)
                    n2594 = local read "FF 2"() -> (→"Frictional Force ( N )" →"Frictional Force ( N )":dbl)
                    n2595 = Build Path(base path=w3180, name or relative path=w3181) -> (appended path=w3176:path)
                    n2596 = flat-sequence {
                      tunnel: w3170 -> [w3236]
                      tunnel: [w3235] -> w3168
                      tunnel: w3167 -> [w3233]
                      tunnel: [w3238] -> w3169
                      tunnel: w3168 -> [w3238]
                      frame #0 {
                        n2597 = call <vilib>:"Mean PtByPt.vi"("x"=w3236, "sample length"="STROKE FILTER", "initialize"=w3233) -> ("mean"=w3235:dbl)  [unwired: 1 in, 1 out]
                      }
                      frame #1 {
                        "STROKE Initialize" <- FALSE ("STROKE Initialize")
                      }
                    }
                    n2598 = local read "COF 2"() -> (w3190:dbl)
                    "Coefficient of Friction" <- w3190
                    "COF 4" <- w3190
                    "Coefficient of Friction" <- w3190
                    n2599 = local read "TEMP"() -> (w3193:dbl)
                    "Temperature ( Deg C )" <- w3193
                    n2600 = local read "Humidity ( %RH )"() -> (w3192:dbl)
                    "Humidity ( %RH ) 2" <- w3192
                    n2601 = local read "Frequency ( Hz )"() -> (w3199:dbl)
                    n2602 = local read "LVDT STROKE DISPLAY"() -> (w3171:dbl)
                    n2603 = local read "Elapsed time"() -> (w3224:dbl)
                    n2604 = local read "AIR TEMP"() -> (w3197:dbl)
                    n2605 = local read "PID-out"() -> (w3202:dbl)
                    n2606 = local write "Temperature ( Deg C )"(w3193) -> ()
                    n2607 = Number To Fractional String(number=w3171, width (-)=i16 9 ("precision (6)"), precision (6)=i16 6) -> (F-format string=w3217:string)  [unwired: 1 in]
                    n2608 = Number To Fractional String(number=w3197, width (-)=i16 9 ("precision (6)"), precision (6)=i16 3) -> (F-format string=w3216:string)  [unwired: 1 in]
                    n2609 = Number To Fractional String(number=w3193, width (-)=i16 9 ("precision (6)"), precision (6)=i16 3) -> (F-format string=w3213:string)  [unwired: 1 in]
                    n2610 = Number To Fractional String(number=w3192, width (-)=i16 9 ("precision (6)"), precision (6)=i16 3) -> (F-format string=w3210:string)  [unwired: 1 in]
                    n2611 = Number To Fractional String(number=0.0, width (-)=i16 9 ("precision (6)"), precision (6)=i16 3) -> (F-format string=w3207:string)  [unwired: 1 in]
                    n2612 = Number To Fractional String(number=w3202, width (-)=i16 9 ("precision (6)"), precision (6)=i16 3) -> (F-format string=w3203:string)  [unwired: 1 in]
                    n2613 = Number To Fractional String(number=w3199, width (-)=i16 9 ("precision (6)"), precision (6)=i16 3) -> (F-format string=w3198:string)  [unwired: 1 in]
                    n2614 = Number To Fractional String(number=w3190, width (-)=i16 9 ("precision (6)"), precision (6)=i16 6) -> (F-format string=w3225:string)  [unwired: 1 in]
                    n2615 = Number To Fractional String(number=w3224, width (-)=i16 14 ("precision (6)"), precision (6)=i16 3) -> (F-format string=w3226:string)  [unwired: 1 in]
                    n2616 = Bundle("y"=1.02, "LVDT STROKE DISPLAY"=w3171, "y"=0.98) -> (w3191:T30)  [unwired: 1 in]
                    n2617 = Number To Fractional String(number="Ambient Humidity :", width (-)=i16 9 ("precision (6)"), precision (6)=i16 6) -> (F-format string=w3183:string)  [unwired: 1 in]
                    n2618 = local read "RUN"() -> (w3189:bool)
                    n2619 = case shown="True" w3189 {
                      tunnel: w3191 -> [_ w3242]
                      tunnel: w3171 -> [_ w3241]
                      tunnel: w3171 -> [_ w3239]
                      tunnel: w3171 -> [_ w3240]
                      frame False {
                      }
                      frame True {
                        "Stroke ( mm )" <- w3242
                        "Stroke ( mm )" <- w3242
                        "Stroke 4" <- w3241
                        "Stroke 3" <- w3239
                        "Stroke 2" <- w3240
                        "measured_stroke" <- w3239
                      }
                    }
                    n2620 = Concatenate Strings(w3226, w3185, w3225, w3185, w3217, w3185, w3216, w3185, w3213, w3185, w3210, w3185, w3207, w3185, w3203, w3185, w3198, w3185, w3183, "\r") -> (w3223:string)
                    n2621 = call <vilib>:"Write Characters To File.vi"("append to file? (new file:F)"=TRUE, "character string"=w3223, "file path (dialog if empty)"=w3176) -> ()  [unwired: 2 in, 1 out]
                    "refresh flag" <- TRUE ("refresh flag")
                    "LVDT STROKE Actual" <- w3169
                  }
                }
                n2622 = case shown="True" w3086 {
                  tunnel: w3096 -> [_ w3122]
                  tunnel: w3101 -> [_ w3132]
                  tunnel: [0.0 w3128] -> _
                  tunnel: w3095 -> [_ w3127]
                  tunnel: [0.0 w3126] -> _
                  tunnel: w3085 -> [_ w3126]
                  tunnel: w3099 -> [w3115 _]
                  frame False {
                    n2623 = local write "acq timer"(w3115) -> ()
                    n2624 = local write "Test Duration Status"(0.0 ("Test Duration Status")) -> ()
                  }
                  frame True {
                    n2625 = local read "Set Hz"() -> (w3129:dbl)
                    n2626 = local write "Elapsed time"(w3122) -> ()
                    n2627 = local read "test time"() -> (w3121:dbl)
                    n2628 = Multiply(x=w3132, y=w3129) -> (x*y=w3131:dbl)
                    n2629 = case shown="False" w3127 {
                      tunnel: w3131 -> [w3133 _]
                      tunnel: [w3133 1.0] -> w3128
                      frame False {
                        n2630 = local write "Cycles elapsed"(w3133) -> ()
                      }
                      frame True {
                      }
                    }
                    n2631 = Greater?(x=w3122, y=w3121) -> (0:w3130:bool)
                    n2632 = Subtract(x=w3121, y=w3122) -> (x-y=w3120:dbl)
                    n2633 = Multiply(x=w3120, y=60.0) -> (x*y=w3119:dbl)
                    n2634 = local write "Time Remaining"(w3119) -> ()
                    n2635 = local write "Remaining Time"(w3119) -> ()
                    n2636 = case shown="True" w3130 {
                      frame False {
                      }
                      frame True {
                        n2637 = stacked-sequence {
                          frame #0 {
                            w3138 = T19."Enabled" ("Disabled")
                            w3137 = FALSE ("TEST FILE NAM,E SAVED")
                            w3139 = "" ("FILE")
                            w3140 = TRUE ("Visible")
                            n2638 = local write "RUN"(FALSE ("OK Button 2")) -> ()
                            n2639 = local write "Heater Button"(FALSE ("Heater Button")) -> ()
                            n2640 = local write "Auto Start Test"(FALSE ("Auto Start Test")) -> ()
                            n2641 = local write "TestCompFlg"(TRUE ("StpFlg")) -> ()
                            n2642 = local read "Humidity ( %RH )"() -> (→"Rh After":dbl)
                            n2643 = property on="STOP 2" class="Bool (strict)"("Disabled"=u8 0) -> ()  [unwired: 2 in, 2 out]
                            n2644 = local read "EVENT LOG"() -> (w3145:string)
                            n2645 = call "Event Log.vi"("Content"="Test Completed", "EVENT LOG"=w3145) -> ("EVENT LOG"=w3144:string)  [unwired: 8 in, 1 out]
                            n2646 = property on="RUN" class="Bool (strict)"("Visible"=w3140) -> ()  [unwired: 2 in, 2 out]
                            n2647 = property on="Auto Start Test" class="Bool (strict)"("Visible"=w3140) -> ()  [unwired: 2 in, 2 out]
                            n2648 = local write "Batch Ref Num :"(w3139) -> ()
                            n2649 = local write "FILE"(w3139) -> ()
                            n2650 = local write "EVENT LOG"(w3144) -> ()
                            n2651 = local write "TEST FILE NAM,E SAVED"(w3137) -> ()
                            n2652 = local write "Fuel Discription :"(w3139) -> ()